vi "Dresden R2R Sputter 03.02.2018 IY24.vi"() -> ()   [LabVIEW 2009] (continued)
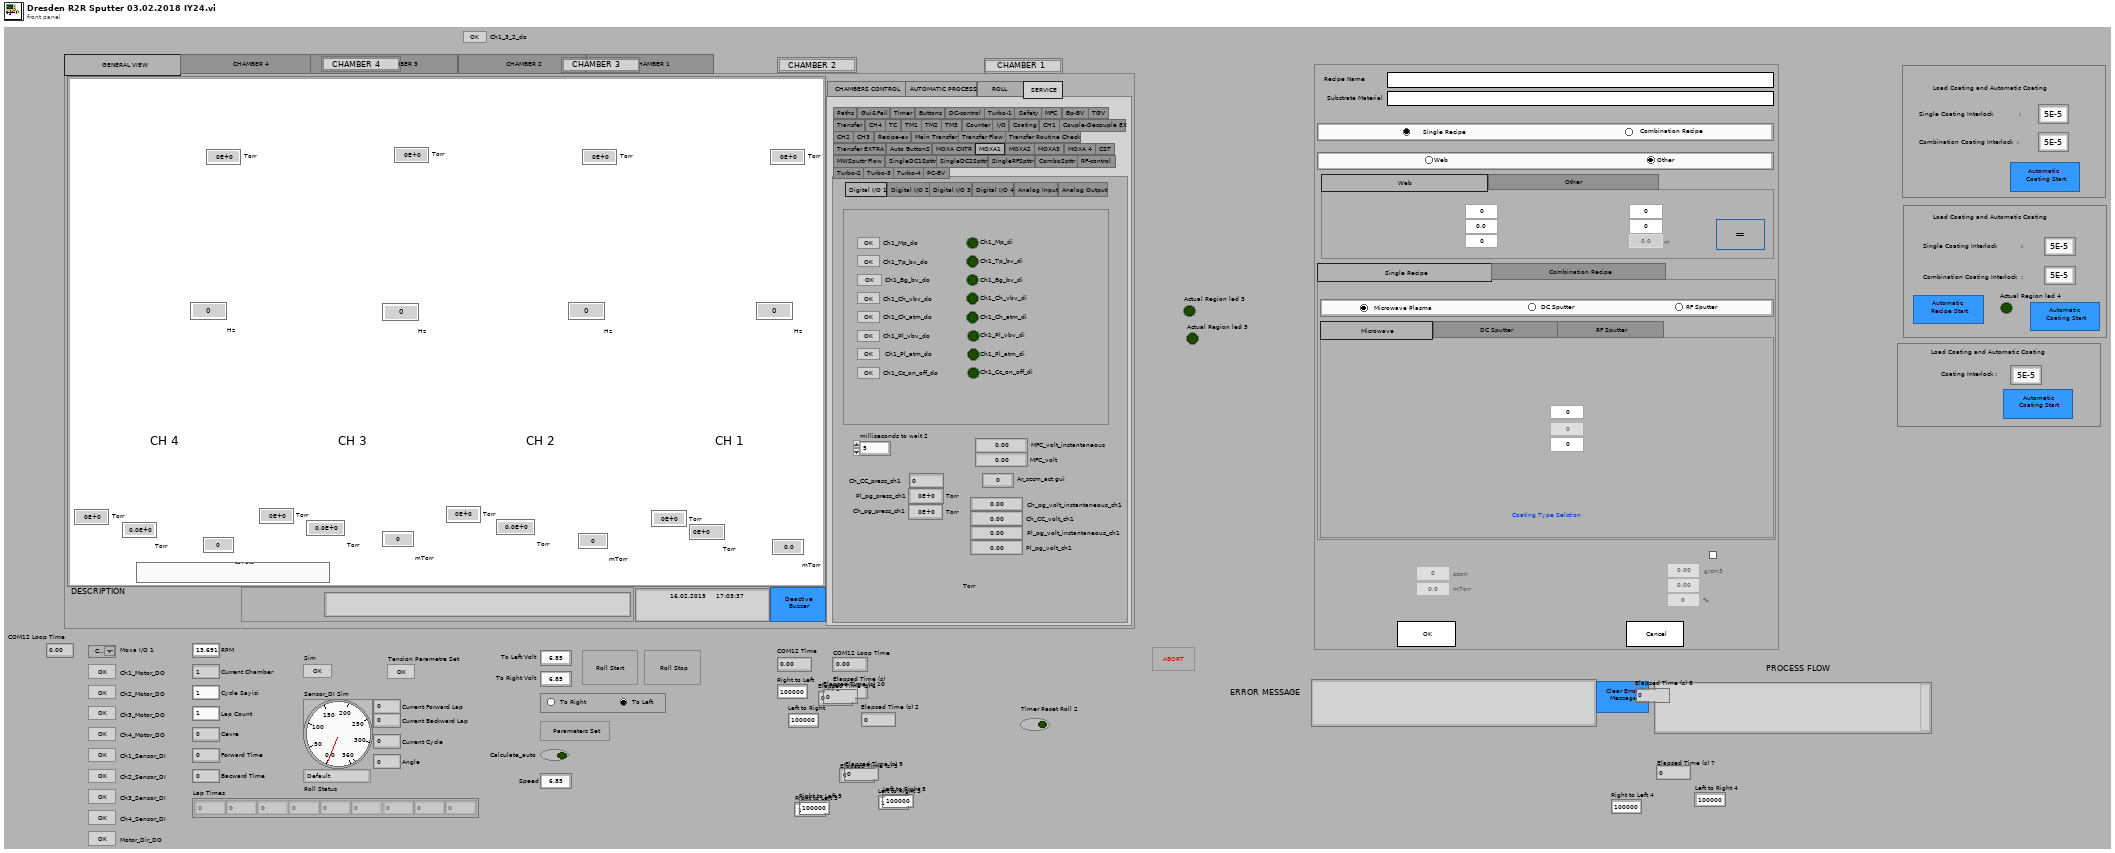
[diagram p1: front panel]
types:
  T1 = typedef "Roll_StatusT.ctl" = enum16{"Default", "Initiate", "Transfer", "Start", "Home", "HomeP", "Forward", "Pause", "Backward", "Stop", "Security"}
  T2 = enum32{"Single Recipe                                                                         ", "Combination Recipe                                                              "}
  T3 = enum32{"Microwave Plasma", "DC Sputter", "RF Sputter"}
  T4 = enum32{"Microwave                                          ", "DC Sputter                                                 ", "RF Sputter                                       "}
  T5 = enum32{"Web                                                                                    ", "Other                                                                                    "}
  T6 = enum32{"  GENERAL VIEW                                   ", "     CHAMBER 4                                             ", "              CHAMBER 3                                              ", " CHAMBER 2                                                ", " CHAMBER 1                                                "}
  T7 = enum32{"CHAMBERS CONTROL    ", "AUTOMATIC PROCESS", "ROLL             ", "SERVICE    "}
  T8 = enum32{"CHAMBER 4      ", "CHAMBER 3       ", "CHAMBER 2       ", "CHAMBER 1         "}
  T9 = enum32{"PUMP & SHUTDOWN CONTROL               ", "PROCESS FLOW                    "}
  T10 = enum32{"Pumping(ch4>0.9 torr)", "Pumping(ch4<0.9 torr)", "Shut Down "}
  T11 = enum32{"Pumping(ch3>0.9 torr)", "Pumping(ch3<0.9 torr)   ", "Shut Down       "}
  T12 = enum32{"Pumping(CH2>0.9 Torr)     ", "Pumping(ch2<0.9 torr)", "Shut Down    "}
  T13 = enum32{"Pumping(CH1>0.9 Torr ", "Pumping(CH1<0.9Torr)    ", "Shut Down       "}
  T14 = enum32{"Chamber I", "Chamber 2", "Chamber 3", "Chamber 4"}
  T15 = enum32{"Full Foil              ", "Specified Length of Foil "}
  T16 = enum32{"Left to Right                ", "Right to Left                  "}
  T17 = enum32{"Paths", "Gui&Fail", "Timer", "Buttons", "DC-control", "Turbo-1", "Safety", "MFC", "Bp-BV", "TGV", "Transfer", "CH4", "TC", "TM1", "TM2", "TM3", "Counter", "I/O", "Coating", "CH1", "Couple-Decouple EX", "CH2", "CH3", "Recipe-ex", "Main Transfer", "Transfer Flow", "Transfer Routine Check", "Transfer EXTRA", "Auto ButtonS", "MOXA CNTR", "MOXA1", "MOXA2", "MOXA3", "MOXA 4", "CST", "MWSputtr Flow", "SingleDC1Spttr", "SingleDC2Spttr", "SingleRFSpttr", "ComboSpttr", "RF-control", "Turbo-2", "Turbo-3", "Turbo-4", "PC-BV"}
  T18 = enum32{"    Page 1        ", "      Page 2        ", "         Page 3        "}
  T19 = enum32{"             Page 1            ", "           Page 2            ", "          Page 3           "}
  T20 = enum32{"Paths", "Gui&fail", "Timer", "Moxa-Ch4", "Buttons", "Automatic Procedure Process Flow", "Auto Pump", "Auto Shutdown", "Transfer4_3"}
  T21 = enum32{"TC1", "TC 2", "Rolling Parameters", "Test"}
  T22 = enum32{"Paths", "Gu&Fail", "Timer", "Moxa-Ch1", "Buttons", "Auto Pump", "Auto shutdown"}
  T23 = enum32{"Paths", "Gui&Fail", "Timer", "Moxa-Ch2", "Buttons", "Auto Pump", "Auto shutdown", "transfer2-3"}
  T24 = enum32{"Paths", "Gui&Fail", "Timer", "Moxa-Ch2", "Buttons", "Auto Pump", "Auto Shut Down", "transfer"}
  T25 = enum32{"Transfer CH1-CH2", "Transfer CH2-CH3 ", "Transfer CH3-CH4", "Transfer CH2-CH1", "Transfer CH3-CH2", "Transfer CH4-CH3"}
  T26 = enum32{"Digital I/O 1", "Digital I/O 2", "Analog Output"}
  T27 = enum32{"Digital I/O 1", "Digital I/O 2", "Digital I/O 3", "Digital I/O 4", "Analog Input", "Analog Output"}
  T28 = enum32{"MANUAL RF COATING CONTROL                                         "}
  T29 = enum32{"RF Power Supply Control", "  Ramp Timer", "Pulsing ", "Capacitor"}
  T30 = enum32{"MANUAL DC COATING CONTROL                                   ..."}
  T31 = enum32{"DC Power Supply Control           ", "Ramp Timer                "}
  T32 = enum32{"DC Power Supply Control   ", "Ramp Timer                     "}
  T33 = enum32{"MANUAL MICROWAVE PLASMA CONTROL                            "}
  T34 = typedef "imagedata.ctl" = cluster{"image type":i32, "image depth":i32, "image":u8[], "mask":u8[], "colors":u32[], "Rectangle":cluster{"left":i16, "top":i16, "right":i16, "bottom":i16}}
  T35 = cluster{"Font Name:":string, "Size":i16, "Strikeout?":bool, "Italic?":bool, "Underline?":bool, "Outline?":bool, "Shadow?":bool, "Bold?":bool}
  T36 = enum16{"User-specified Font", "Application Font", "System Font", "Dialog Font"}
  T37 = typedef "LVMouseTypeDef.ctl" = cluster{"Mouse Position":cluster{"X":i32, "Y":i32}, "Mouse Modifiers":cluster{"Button Down":bool, "Shift Mod":bool, "Menu Mod":bool, "Option Mod":bool}}
  T38 = cluster{"Button Down":bool, "Shift Mod":bool, "Menu Mod":bool, "Option Mod":bool}
  T39 = cluster{"Mode":enum16{"RTU", "ASCII"}, "Slave Address":u8}
  T40 = enum16{"Left Button", "Center Button", "Right Button", "Window Close"}
diagram:
  w2 = data[3B] items=["Default", "Initiate", "Transfer", "Start", "Home", "HomeP", "Forward", "Pause", "Backward", "Stop", "Security"] ("Roll Status")
  w22 = data[3B] items=["RTU", "ASCII"] ("Mode")
  w20 = data[3B] items=["None", "Odd", "Even", "Mark", "Space"] ("Parity")
  (unwired) i32? 19200 ("Baud Rate")
  w28 = data[3B] items=["RTU", "ASCII"] ("Mode")
  w30 = data[3B] items=["None", "Odd", "Even", "Mark", "Space"] ("Parity")
  w750 = data[3B] items=["RTU", "ASCII"] ("Mode")
  w752 = data[3B] items=["None", "Odd", "Even", "Mark", "Space"] ("Parity")
  w766 = data[3B] items=["RTU", "ASCII"] ("Mode")
  w764 = data[3B] items=["None", "Odd", "Even", "Mark", "Space"] ("Parity")
  w767 = data[3B] items=["RTU", "ASCII"] ("Mode")
  w769 = data[3B] items=["None", "Odd", "Even", "Mark", "Space"] ("Parity")
  w780 = data[3B] items=["RTU", "ASCII"] ("Mode")
  w778 = data[3B] items=["None", "Odd", "Even", "Mark", "Space"] ("Parity")
  w787 = data[3B] items=["RTU", "ASCII"] ("Mode")
  w785 = data[3B] items=["None", "Odd", "Even", "Mark", "Space"] ("Parity")
  w792 = data[3B] items=["RTU", "ASCII"] ("Mode")
  w794 = data[3B] items=["None", "Odd", "Even", "Mark", "Space"] ("Parity")
  w821 = i16? 1 items=["None", "Odd", "Even", "Mark", "Space"] ("parity (0:none)")
  w825 = i16? 2 items=["None", "Odd", "Even", "Mark", "Space"] ("parity (0:none)")
  w834 = i16? 1 items=["None", "Odd", "Even", "Mark", "Space"] ("parity (0:none)")
  # "Timer"
  # "Elapsed Time Array"
  # "Status"
  # "Chamber No"
  # "*Initiate\nAmac: Baslangic degerlerinin okuyor ve start val bekliyor.\nBulundugu camber degerini okuyor. (1-4)\nLap sayisini okuyor.\nCycle sayisini okuyor.\n\nSistem hep soldan saga sarma yapabiliyor.\n\nStart val degerini okuyan loop yapıyor.\nStart val 1 olmasi ile Start state'e gidiyor.\n\n*Start State\nAmac: Motoru calıstırmak. \nMotoru Calistiriyor.\nHome state'e gidiyor.\n\n*Home State\nAmac: Belirli bir ref noktadan prosesi baslatmak.\nTam dolu yarim aya girince baslatir.\nDolu yarim aya girince forward state'e gidiyor.\nForward Timer baslatilir.\n\n*Forward State\nBaslangicta dolu yarim ayin basindan sonuna ilerler ve bosa cikar.\nIlk tur icinde once bosa cikar ve\nDolu yarim aya tekrar girince tur atmis olur.\nTur atlayinca Lap Sayisini 1 azaltir. Back Lap sayisini 1 arttirir.\nBack tur sayisi ilk tur ile birlikte 2 olur. Cunku Geri gidiste, \ntur atmadan ilk bosa dususu kompanse etmek gerekmektedir.\nLap sayisi kalan degeri 0 olunca Pause State'e gider.\nLap Times'a Forward Lap Time kayit edilir.\n\n*Backward State\nBaslangicta dolu yarim ayin hemen basindan geri gider ve bosa cikar,\nİlk bosa cikis tam tur olmadigindan deger back tur degeri 2 den 1 olur.\nIlk tur icinde once bosata ilerler ve dolu tarafa gecer.\nDolu yarim ay tekrar bitince geri tur atmis olur.\nTur atlayinca Back Lap sayisini 1 azalir.\nBack Lap sayisi kalan degeri 0 olunca Cycle degeri 1 azalir.\nCycle sayisi degeri 0 olursa Stop State'e yoksa Pause State'e gider.\nLap Times'a Backward Lap Time kayit edilir.\n\n*Pause State\nMotorlarin tamamina dur komutu yollanir.\n1 saniye beklenir.\nYon degistirilir.\nLap Times'a Pause yi gosteren 0 degeri kayit edilir.\nTension Parametre Set Yollanir.\nMotor calıstırılır.\nBackward veya Forward Timer baslatilir."
  # "Moxa R1212 uzerinde \nDI starting adresi 0 ve quantity 16 adet yapılabilir.\nDO starting adres 320 ve quantity girmeye gerekyok.\n\nMoxa manuelinde \n1 nolu adres DI0 value demek.\n321 nolu adres DO_0 value demek.\nLabview, Manuele adresinden 1 eksik degerler istiyor.\n \nVaksis programlarında DI starting adres 8 olarak secilmis. (8 secilmesinin nedeni ilk 8 adresin jumperlar ile DO DI yapilabilir adresler olmasi ve bunların DO olarak kullanılması olabilir.)"
  # "Moxa R1212 uzerinde \n8 adet DI \n8 adet DO bulunmaktadir. \nDO jumper ile DI'ye donusturulebilmektedir."
  # "Back Tur"
  # "Cycle"
  # "Forward Tur"
  # "Speed"
  # "right to left 4/5 true 2/2 actual region led"
  # "Gui & Text"
  # "Digital & Analog Inputs / Outputs"
  # "TRANSFER PROCESS"
  n1 = while {
    stop <- FALSE stop-if-true
    n2 = Wait Until Next ms Multiple(millisecond multiple=u32 300) -> ()  [unwired: 1 out]
    n3 = local read "Start_up_ch2"() -> (w852:bool)
    n4 = local read "Start_up_ch3"() -> (w847:bool)
    n5 = local read "Start_up_ch4"() -> (w844:bool)
    n6 = local read "Start_up_ch1"() -> (w855:bool)
    n7 = case shown="True" w852 {
      frame #0 {
      }
      frame #1 {
        n8 = local read "Ch2_pressure2"() -> (→"Pressure_time_graph_ch2":dbl)
        n9 = Wait (ms)(milliseconds to wait=u32 1000) -> ()  [unwired: 1 out]
      }
    }
    n10 = case shown="True" w847 {
      frame #0 {
      }
      frame #1 {
        n11 = local read "Ch3_pressure2"() -> (→"Pressure_time_graph_ch3":dbl)
        n12 = Wait (ms)(milliseconds to wait=u32 1000) -> ()  [unwired: 1 out]
      }
    }
    n13 = case shown="True" w844 {
      frame #0 {
      }
      frame #1 {
        n14 = local read "Ch4pressure"() -> (→"Pressure_time_graph_ch4":dbl)
        n15 = Wait (ms)(milliseconds to wait=u32 1000) -> ()  [unwired: 1 out]
      }
    }
    n16 = case shown="True" w855 {
      frame #0 {
      }
      frame #1 {
        n17 = local read "Ch1_pressure 2"() -> (→"Pressure_time_graph_ch1":dbl)
        n18 = Wait (ms)(milliseconds to wait=u32 1000) -> ()  [unwired: 1 out]
      }
    }
    n19 = feedback #1() -> (w851:bool)  [unwired: 1 in]
    n20 = feedback #2() -> (w856:bool)  [unwired: 1 in]
    n21 = feedback #3() -> (w848:bool)  [unwired: 1 in]
    n22 = feedback #4() -> (w843:bool)  [unwired: 1 in]
    n23 = case shown="True" w852 {
      tunnel: [TRUE FALSE] -> w850
      tunnel: w851 -> [_ w904]
      frame #0 {
      }
      frame #1 {
        n24 = call "Elapsed Time126"("Reset"=w904) -> ("Elapsed Time (s)"=→"Auto_pump_time_ch2" →"Graph_pumping_time_ch2":dbl)  [unwired: 11 in, 7 out]
      }
    }
    n25 = case shown="True" w855 {
      tunnel: [TRUE FALSE] -> w857
      tunnel: w856 -> [_ w920]
      frame #0 {
      }
      frame #1 {
        n26 = call "Elapsed Time101"("Reset"=w920) -> ("Elapsed Time (s)"=→"Auto_pump_time_ch1" →"Graph_pumping_time_ch1":dbl)  [unwired: 11 in, 7 out]
      }
    }
    n27 = case shown="True" w847 {
      tunnel: [TRUE FALSE] -> w849
      tunnel: w848 -> [_ w888]
      frame #0 {
      }
      frame #1 {
        n28 = call "Elapsed Time128"("Reset"=w888) -> ("Elapsed Time (s)"=→"Auto_pump_time_ch3" →"Graph_pumping_time_ch3":dbl)  [unwired: 11 in, 7 out]
      }
    }
    n29 = case shown="True" w844 {
      tunnel: [TRUE FALSE] -> w842
      tunnel: w843 -> [_ w872]
      frame #0 {
      }
      frame #1 {
        n30 = call "Elapsed Time137"("Reset"=w872) -> ("Elapsed Time (s)"=→"Auto_pump_time_ch4" →"Graph_pumping_time_ch4":dbl)  [unwired: 11 in, 7 out]
      }
    }
    n31 = case shown="True" w852 {
      frame #0 {
      }
      frame #1 {
        n32 = local read "Graph_pumping_time_ch2"() -> (w899:dbl)
        n33 = Divide(x=w899, y=60.0 ("X Scale.Range:Maximum")) -> (x/y=w900:dbl)
        n34 = Increment(x=w900) -> (x+1=w898:dbl)
        n35 = property on="Pressure_time_graph_ch2" class="WFChart (strict)"("XScale.Maximum"=w898, "XScale.Minimum"=0.0 ("X Scale.Range:Minimum")) -> ()  [unwired: 2 in, 2 out]
        n36 = property on="Pressure_time_graph_ch2" class="WFChart (strict)"("YScale.Maximum"=1000.0 ("Y Scale.Range:Maximum"), "YScale.Minimum"=5e-08 ("Y Scale.Range:Minimum")) -> ()  [unwired: 2 in, 2 out]
        n37 = property on="Pressure_time_graph_ch2" class="WFChart (strict)"("XScale.Multiplier"=0.0166 ("X Scale.Offset and Multiplier:Multiplier 2")) -> ()  [unwired: 2 in, 2 out]
      }
    }
    n38 = case shown="True" w855 {
      frame #0 {
      }
      frame #1 {
        n39 = local read "Graph_pumping_time_ch1"() -> (w915:dbl)
        n40 = Divide(x=w915, y=60.0 ("X Scale.Range:Maximum")) -> (x/y=w916:dbl)
        n41 = Increment(x=w916) -> (x+1=w914:dbl)
        n42 = property on="Pressure_time_graph_ch1" class="WFChart (strict)"("XScale.Maximum"=w914, "XScale.Minimum"=0.0 ("X Scale.Range:Minimum")) -> ()  [unwired: 2 in, 2 out]
        n43 = property on="Pressure_time_graph_ch1" class="WFChart (strict)"("YScale.Maximum"=1000.0 ("Y Scale.Range:Maximum"), "YScale.Minimum"=5e-08 ("Y Scale.Range:Minimum")) -> ()  [unwired: 2 in, 2 out]
        n44 = property on="Pressure_time_graph_ch1" class="WFChart (strict)"("XScale.Multiplier"=0.0166 ("X Scale.Offset and Multiplier:Multiplier 2")) -> ()  [unwired: 2 in, 2 out]
      }
    }
    n45 = case shown="True" w847 {
      frame #0 {
      }
      frame #1 {
        n46 = local read "Graph_pumping_time_ch3"() -> (w883:dbl)
        n47 = Divide(x=w883, y=60.0 ("X Scale.Range:Maximum")) -> (x/y=w884:dbl)
        n48 = Increment(x=w884) -> (x+1=w882:dbl)
        n49 = property on="Pressure_time_graph_ch3" class="WFChart (strict)"("XScale.Maximum"=w882, "XScale.Minimum"=0.0 ("X Scale.Range:Minimum")) -> ()  [unwired: 2 in, 2 out]
        n50 = property on="Pressure_time_graph_ch3" class="WFChart (strict)"("YScale.Maximum"=1000.0 ("Y Scale.Range:Maximum"), "YScale.Minimum"=5e-08 ("Y Scale.Range:Minimum")) -> ()  [unwired: 2 in, 2 out]
        n51 = property on="Pressure_time_graph_ch3" class="WFChart (strict)"("XScale.Multiplier"=0.0166 ("X Scale.Offset and Multiplier:Multiplier 2")) -> ()  [unwired: 2 in, 2 out]
      }
    }
    n52 = case shown="True" w844 {
      frame #0 {
      }
      frame #1 {
        n53 = local read "Graph_pumping_time_ch4"() -> (w867:dbl)
        n54 = Divide(x=w867, y=60.0 ("X Scale.Range:Maximum")) -> (x/y=w868:dbl)
        n55 = Increment(x=w868) -> (x+1=w866:dbl)
        n56 = property on="Pressure_time_graph_ch4" class="WFChart (strict)"("XScale.Maximum"=w866, "XScale.Minimum"=0.0 ("X Scale.Range:Minimum")) -> ()  [unwired: 2 in, 2 out]
        n57 = property on="Pressure_time_graph_ch4" class="WFChart (strict)"("YScale.Maximum"=1000.0 ("Y Scale.Range:Maximum"), "YScale.Minimum"=5e-08 ("Y Scale.Range:Minimum")) -> ()  [unwired: 2 in, 2 out]
        n58 = property on="Pressure_time_graph_ch4" class="WFChart (strict)"("XScale.Multiplier"=0.0166 ("X Scale.Offset and Multiplier:Multiplier 2")) -> ()  [unwired: 2 in, 2 out]
      }
    }
    n59 = case shown="True" "Show_graph_ch2" {
      frame #0 {
        n60 = property on="Graph_tab_ch2" class="TabCtl (strict)"("Visible"=TRUE) -> ()  [unwired: 2 in, 2 out]
      }
      frame #1 {
        n61 = property on="Graph_tab_ch2" class="TabCtl (strict)"("Visible"=FALSE) -> ()  [unwired: 2 in, 2 out]
      }
    }
    n62 = case shown="True" "Show_graph_ch1" {
      frame #0 {
        n63 = property on="Graph_tab_ch1" class="TabCtl (strict)"("Visible"=TRUE) -> ()  [unwired: 2 in, 2 out]
      }
      frame #1 {
        n64 = property on="Graph_tab_ch1" class="TabCtl (strict)"("Visible"=FALSE) -> ()  [unwired: 2 in, 2 out]
      }
    }
    n65 = case shown="True" "Show_graph_ch3" {
      frame #0 {
        n66 = property on="Graph_tab_ch3" class="TabCtl (strict)"("Visible"=TRUE) -> ()  [unwired: 2 in, 2 out]
      }
      frame #1 {
        n67 = property on="Graph_tab_ch3" class="TabCtl (strict)"("Visible"=FALSE) -> ()  [unwired: 2 in, 2 out]
      }
    }
    n68 = case shown="True" "Show_graph_ch4" {
      frame #0 {
        n69 = property on="Graph_tab_ch4" class="TabCtl (strict)"("Visible"=TRUE) -> ()  [unwired: 2 in, 2 out]
      }
      frame #1 {
        n70 = property on="Graph_tab_ch4" class="TabCtl (strict)"("Visible"=FALSE) -> ()  [unwired: 2 in, 2 out]
      }
    }
  }
  n71 = while {
    stop <- FALSE stop-if-true
    n72 = local read "Semi"() -> (w924:bool)
    n73 = Wait Until Next ms Multiple(millisecond multiple=u32 300) -> ()  [unwired: 1 out]
    n74 = feedback #5() -> (w926:bool)  [unwired: 1 in]
    n75 = case shown="True" w924 {
      tunnel: w926 -> [_ w946]
      tunnel: [TRUE FALSE] -> w925
      frame #0 {
      }
      frame #1 {
        w930 = FALSE
        w932 = FALSE
        n76 = call "Elapsed Time99"("Reset"=w946) -> ("Elapsed Time (s)"=w933:dbl)  [unwired: 11 in, 7 out]
        n77 = In Range and Coerce(upper limit=2.3, x=w933, lower limit=2.0) -> (In Range?=w943:bool)  [unwired: 1 out]
        n78 = In Range and Coerce(upper limit=4.3, x=w933, lower limit=4.0) -> (In Range?=w942:bool)  [unwired: 1 out]
        n79 = In Range and Coerce(upper limit=6.3, x=w933, lower limit=6.0) -> (In Range?=w937:bool)  [unwired: 1 out]
        n80 = In Range and Coerce(upper limit=11.3, x=w933, lower limit=11.0) -> (In Range?=w936:bool)  [unwired: 1 out]
        n81 = In Range and Coerce(upper limit=0.3, x=w933, lower limit=0.0) -> (In Range?=w931:bool)  [unwired: 1 out]
        n82 = disable-structure shown="Disabled" {
          disable-tunnel: w943 -> [w953 _]
          disable-tunnel: w942 -> [w952 _]
          disable-tunnel: w937 -> [w951 _]
          disable-tunnel: w931 -> [w950 _]
          frame #0 {
            n83 = case shown="True" w950 {
              frame #0 {
              }
              frame #1 {
                w958 = FALSE
                w959 = FALSE
                w960 = FALSE
                w961 = TRUE
                w962 = FALSE
                w963 = TRUE
                w964 = TRUE ("Cnt_Do_Buzzer")
                w965 = FALSE
                n84 = local write "Casette_servo_start/stop_do"(w965) -> ()
                n85 = local write "Tension_controllers_start/stop_do"(w965) -> ()
                n86 = local write "Security_cancel_ch1"(w963) -> ()
                n87 = local write "Security_cancel_ch2"(w963) -> ()
                n88 = local write "Security_cancel_ch3"(w963) -> ()
                n89 = local write "Security_cancel_ch4"(w963) -> ()
                n90 = local write "Ch1_Tp_bv_do"(w962) -> ()
                n91 = local write "Ch1_Bg_bv_do"(w962) -> ()
                n92 = local write "Ch1_Ch_vbv_do"(w962) -> ()
                n93 = local write "Ch1_Pl_vbv_do"(w962) -> ()
                n94 = local write "Ch1_Cc_on_off_do"(w962) -> ()
                n95 = local write "Ch1_Sov_Ar_do"(w962) -> ()
                n96 = local write "Ch1_SRV_start_stop_do"(w962) -> ()
                n97 = local write "Ch1_TGV_control_do"(w962) -> ()
                n98 = local write "Pc_bv1_auto_close"(w961) -> ()
                n99 = local write "Tp1_auto_stop"(w961) -> ()
                n100 = local write "Ch3_Tp_bv_do"(w959) -> ()
                n101 = local write "Ch3_Bg_bv_do"(w959) -> ()
                n102 = local write "Ch3_Ch_vbv_do"(w959) -> ()
                n103 = local write "Ch3_Pl_vbv_do"(w959) -> ()
                n104 = local write "Ch3_Cc_on_off_do"(w959) -> ()
                n105 = local write "Ch3_Sov_Ar_do"(w959) -> ()
                n106 = local write "Ch3_SRV_start_stop_do"(w959) -> ()
                n107 = local write "Ch3_TGV_control_do"(w959) -> ()
                n108 = local write "Cnt_Do_Buzzer"(w964) -> ()
                n109 = local write "Ar_auto_set_zero_ch1"(w964) -> ()
                n110 = local write "Dc_auto_off"(w964) -> ()
                n111 = local write "RF_auto_off"(w964) -> ()
                n112 = local write "MW1_off"(w964) -> ()
                n113 = local write "Test_stop"(w964) -> ()
                n114 = local write "Ch2_Tp_bv_do"(w960) -> ()
                n115 = local write "Ch2_Bg_bv_do"(w960) -> ()
                n116 = local write "Ch2_Ch_vbv_do"(w960) -> ()
                n117 = local write "Ch2_Pl_vbv_do"(w960) -> ()
                n118 = local write "Ch2_Cc_on_off_do"(w960) -> ()
                n119 = local write "Ch2_Sov_Ar_do"(w960) -> ()
                n120 = local write "Ch2_SRV_start_stop_do"(w960) -> ()
                n121 = local write "Ch2_TGV_control_do"(w960) -> ()
                n122 = local write "Ch4_Tp_bv_do"(w958) -> ()
                n123 = local write "Ch4_Bg_bv_do"(w958) -> ()
                n124 = local write "Ch4_Ch_vbv_do"(w958) -> ()
                n125 = local write "Ch4_Pl_vbv_do"(w958) -> ()
                n126 = local write "Ch4_Cc_on_off_do"(w958) -> ()
                n127 = local write "Ch4_Sov_Ar_do"(w958) -> ()
                n128 = local write "Ch4_SRV_start_stop_do"(w958) -> ()
                n129 = local write "Ch4_TGV_control_do"(w958) -> ()
              }
            }
            n130 = case shown="True" w952 {
              frame #0 {
              }
              frame #1 {
                w954 = TRUE
                n131 = local write "Pc_bv3_auto_close"(w954) -> ()
                n132 = local write "Tp3_auto_stop"(w954) -> ()
              }
            }
            n133 = case shown="True" w951 {
              frame #0 {
              }
              frame #1 {
                w966 = TRUE
                n134 = local write "Pc_bv4_auto_close"(w966) -> ()
                n135 = local write "Tp4_auto_stop"(w966) -> ()
              }
            }
            n136 = case shown="True" w953 {
              frame #0 {
              }
              frame #1 {
                w955 = TRUE
                w957 = TRUE
                w956 = FALSE
                n137 = local write "Cnt_Dcps_sw1_do"(w956) -> ()
                n138 = local write "Cnt_Dcps_sw2_do"(w956) -> ()
                n139 = local write "Ar_auto_set_zero_ch3"(w957) -> ()
                n140 = local write "MW2_off"(w957) -> ()
                n141 = local write "Pc_bv2_auto_close"(w955) -> ()
                n142 = local write "Tp2_auto_stop"(w955) -> ()
              }
            }
          }
          frame #1 {
          }
        }
        n143 = case shown="True" w936 {
          frame #0 {
          }
          frame #1 {
            w968 = FALSE
            n144 = local write "Security_cancel_ch1"(w968) -> ()
            n145 = local write "Security_cancel_ch2"(w968) -> ()
            n146 = local write "Security_cancel_ch3"(w968) -> ()
            n147 = local write "Security_cancel_ch4"(w968) -> ()
            n148 = local write "Cnt_Do_Buzzer"(w968) -> ()
            n149 = local write "Semi"(w968) -> ()
            n150 = local write "Statue_abort"(w968) -> ()
          }
        }
        n151 = case shown="True" w931 {
          frame #0 {
          }
          frame #1 {
            n152 = local write "Cnt_Do_Buzzer"(TRUE ("Cnt_Do_Buzzer")) -> ()
          }
        }
        n153 = local write "Routine_check_transfer"(w932) -> ()
        n154 = local write "Transfer_ch1_2"(w932) -> ()
        n155 = local write "Transfer_ch2_1"(w932) -> ()
        n156 = local write "Transfer_ch2_3"(w932) -> ()
        n157 = local write "Transfer_ch3_2"(w932) -> ()
        n158 = local write "Transfer_ch3_4"(w932) -> ()
        n159 = local write "Transfer_ch3_4"(w932) -> ()
        n160 = local write "Start_up_ch1"(w932) -> ()
        n161 = local write "Start_up_ch2"(w932) -> ()
        n162 = local write "Start_up_ch3"(w932) -> ()
        n163 = local write "Start_up_ch4"(w932) -> ()
        n164 = local write "Shutdown_ch1"(w932) -> ()
        n165 = local write "Shutdown_ch2"(w932) -> ()
        n166 = local write "Shutdown_ch3"(w932) -> ()
        n167 = local write "Shutdown_ch4"(w932) -> ()
        n168 = local write "Start_coating"(w932) -> ()
        n169 = local write "Start_Coating_MW"(w932) -> ()
        n170 = local write "Start_Coating_Ch4"(w932) -> ()
        n171 = local write "Start_Coating_Ch2"(w932) -> ()
        n172 = local write "Start_Coating_Ch3"(w932) -> ()
        n173 = local write "Casette_servo_start/stop_do"(w930) -> ()
        n174 = local write "Tension_controllers_start/stop_do"(w930) -> ()
        n175 = local write "Automatic Roll"(w930) -> ()
      }
    }
  }
  n176 = stacked-sequence {
    frame #0 {
    }
  }
  n177 = local write "Ch2_TGV_control_do"(T/1 ("Ch2_TGV_control_do")) -> ()
  n178 = stacked-sequence {
    frame #0 {
      w969 = ""
      "Error Message" <- w969
      "system_status" <- "Semi-automatic is active" ("system_statu")
      "final_process_messages" <- w969
    }
  }
  n179 = stacked-sequence {
    frame #0 {
      # "OTHER  BUTTONS"
      n180 = while {
        stop <- i16? 0 stop-if-true
        # "OPEN/CLOSE & START &STOP"
        n181 = stacked-sequence {
          frame #0 {
            n182 = Or(x="Ch1_Mp_start_gui", y="Ch1_Mp_start") -> (x .or. y?=w1776)
            n183 = Or(x="Ch1_Mp_stop_gui", y="Ch1_Mp_stop") -> (x .or. y?=w1775)
            n184 = case shown="True" w1775 {
              frame #0 {
              }
              frame #1 {
                n185 = local read "Ch1_Mp_stop_safety"() -> (w1819)
                n186 = case shown="True" w1819 {
                  frame #0 {
                    n187 = local write "Error Message"("MP can not be stopped.\nReason :                           \n*TP-BV can be open.       " ("Error Message")) -> ()
                  }
                  frame #1 {
                    n188 = stacked-sequence {
                      frame #0 {
                        n189 = local write "Ch1_Mp_do"(i16? 0 ("Ch1_Mp_do")) -> ()
                      }
                      frame #1 {
                        n190 = Wait (ms)(milliseconds to wait=i32? 500) -> ()  [unwired: 1 out]
                      }
                      frame #2 {
                        n191 = local write "Ch1_Pl_atm_do"(i16? 0 ("Ch1_Mp_do")) -> ()
                      }
                      frame #3 {
                        n192 = Wait (ms)(milliseconds to wait=i32? 500) -> ()  [unwired: 1 out]
                      }
                      frame #4 {
                        n193 = local write "Ch1_Pl_vbv_do"(T/1 ("Ch1_Pl_vbv_do")) -> ()
                      }
                    }
                  }
                }
              }
            }
            n194 = case shown="True" w1776 {
              frame #0 {
              }
              frame #1 {
                n195 = local read "Ch1_Mp_start_safety"() -> (w1826)
                n196 = case shown="True" w1826 {
                  frame #0 {
                    n197 = local write "Error Message"("MP can not be started.\nReason:                          \n*PL-VBV can be open. \n   *CH-VBV can be open." ("Error Message")) -> ()
                  }
                  frame #1 {
                    n198 = stacked-sequence {
                      frame #0 {
                        n199 = local write "Ch1_Pl_atm_do"(T/1 ("Ch1_Mp_do")) -> ()
                      }
                      frame #1 {
                        n200 = Wait (ms)(milliseconds to wait=i32? 1000) -> ()  [unwired: 1 out]
                      }
                      frame #2 {
                        n201 = local write "Ch1_Ch_atm_do"(T/1 ("Ch1_Mp_do")) -> ()
                      }
                      frame #3 {
                        n202 = Wait (ms)(milliseconds to wait=i32? 1000) -> ()  [unwired: 1 out]
                      }
                      frame #4 {
                        n203 = local write "Ch1_Mp_do"(T/1 ("Ch1_Mp_do")) -> ()
                      }
                    }
                  }
                }
              }
            }
            n204 = Or(x="Ch2_Mp_start_gui", y="Ch2_Mp_start") -> (x .or. y?=w1773)
            n205 = Or(x="Ch2_Mp_stop_gui", y="Ch2_Mp_stop") -> (x .or. y?=w1774)
            n206 = case shown="True" w1773 {
              frame #0 {
              }
              frame #1 {
                n207 = local read "Ch2_Mp_start_safety"() -> (w1812)
                n208 = case shown="True" w1812 {
                  frame #0 {
                    n209 = local write "Error Message"("MP can not be started.\nReason:*PL-VBV can be open. \n   *CH-VBV can be open." ("Error Message")) -> ()
                  }
                  frame #1 {
                    n210 = stacked-sequence {
                      frame #0 {
                        n211 = local write "Ch2_Pl_atm_do"(T/1 ("Ch1_Mp_do")) -> ()
                      }
                      frame #1 {
                        n212 = Wait (ms)(milliseconds to wait=i32? 1000) -> ()  [unwired: 1 out]
                      }
                      frame #2 {
                        n213 = local write "Ch2_Ch_atm_do"(T/1 ("Ch1_Mp_do")) -> ()
                      }
                      frame #3 {
                        n214 = Wait (ms)(milliseconds to wait=i32? 1000) -> ()  [unwired: 1 out]
                      }
                      frame #4 {
                        n215 = local write "Ch2_Mp_do"(T/1 ("Ch1_Mp_do")) -> ()
                      }
                    }
                  }
                }
              }
            }
            n216 = case shown="True" w1774 {
              frame #0 {
              }
              frame #1 {
                n217 = local read "Ch2_Mp_stop_safety"() -> (w1805)
                n218 = case shown="True" w1805 {
                  frame #0 {
                    n219 = local write "Error Message"("MP can not be stopped.\nReason :*TP-BV can be open." ("Error Message")) -> ()
                  }
                  frame #1 {
                    n220 = stacked-sequence {
                      frame #0 {
                        n221 = local write "Ch2_Mp_do"(i16? 0 ("Ch1_Mp_do")) -> ()
                      }
                      frame #1 {
                        n222 = Wait (ms)(milliseconds to wait=i32? 500) -> ()  [unwired: 1 out]
                      }
                      frame #2 {
                        n223 = local write "Ch2_Pl_atm_do"(i16? 0 ("Ch1_Mp_do")) -> ()
                      }
                      frame #3 {
                        n224 = Wait (ms)(milliseconds to wait=i32? 500) -> ()  [unwired: 1 out]
                      }
                      frame #4 {
                        n225 = local write "Ch2_Pl_vbv_do"(T/1 ("Ch1_Pl_vbv_do")) -> ()
                      }
                    }
                  }
                }
              }
            }
            n226 = Or(x="Ch3_Mp_stop_gui", y="Ch3_Mp_stop") -> (x .or. y?=w1771)
            n227 = Or(x="Ch3_Mp_start_gui", y="Ch3_Mp_start") -> (x .or. y?=w1772)
            n228 = case shown="True" w1772 {
              frame #0 {
              }
              frame #1 {
                n229 = local read "Ch3_Mp_start_safety"() -> (w1798)
                n230 = case shown="True" w1798 {
                  frame #0 {
                    n231 = local write "Error Message"("MP can not be started.\nReason:*PL-VBV can be open. \n   *CH-VBV can be open." ("Error Message")) -> ()
                  }
                  frame #1 {
                    n232 = stacked-sequence {
                      frame #0 {
                        n233 = local write "Ch3_Pl_atm_do"(T/1 ("Ch1_Mp_do")) -> ()
                      }
                      frame #1 {
                        n234 = Wait (ms)(milliseconds to wait=i32? 1000) -> ()  [unwired: 1 out]
                      }
                      frame #2 {
                        n235 = local write "Ch3_Ch_atm_do"(T/1 ("Ch1_Mp_do")) -> ()
                      }
                      frame #3 {
                        n236 = Wait (ms)(milliseconds to wait=i32? 1000) -> ()  [unwired: 1 out]
                      }
                      frame #4 {
                        n237 = local write "Ch3_Mp_do"(T/1 ("Ch1_Mp_do")) -> ()
                      }
                    }
                  }
                }
              }
            }
            n238 = case shown="True" w1771 {
              frame #0 {
              }
              frame #1 {
                n239 = local read "Ch3_Mp_stop_safety"() -> (w1791)
                n240 = case shown="True" w1791 {
                  frame #0 {
                    n241 = local write "Error Message"("MP can not be stopped.\nReason :*TP-BV can be open." ("Error Message")) -> ()
                  }
                  frame #1 {
                    n242 = stacked-sequence {
                      frame #0 {
                        n243 = local write "Ch3_Mp_do"(i16? 0 ("Ch1_Mp_do")) -> ()
                      }
                      frame #1 {
                        n244 = Wait (ms)(milliseconds to wait=i32? 500) -> ()  [unwired: 1 out]
                      }
                      frame #2 {
                        n245 = local write "Ch3_Pl_atm_do"(i16? 0 ("Ch1_Mp_do")) -> ()
                      }
                      frame #3 {
                        n246 = Wait (ms)(milliseconds to wait=i32? 500) -> ()  [unwired: 1 out]
                      }
                      frame #4 {
                        n247 = local write "Ch3_Pl_vbv_do"(T/1 ("Ch1_Pl_vbv_do")) -> ()
                      }
                    }
                  }
                }
              }
            }
            n248 = Or(x="Ch4_Mp_stop_gui", y="Ch4_Mp_stop") -> (x .or. y?=w1754)
            n249 = Or(x="Ch4_Mp_start_gui", y="Ch4_Mp_start") -> (x .or. y?=w1757)
            n250 = case shown="True" w1757 {
              frame #0 {
              }
              frame #1 {
                n251 = local read "Ch4_Mp_start_safety"() -> (w1784)
                n252 = case shown="True" w1784 {
                  frame #0 {
                    n253 = local write "Error Message"("MP can not be started.\nReason:*PL-VBV can be open. \n   *CH-VBV can be open." ("Error Message")) -> ()
                  }
                  frame #1 {
                    n254 = stacked-sequence {
                      frame #0 {
                        n255 = local write "Ch4_Pl_atm_do"(T/1 ("Ch1_Mp_do")) -> ()
                      }
                      frame #1 {
                        n256 = Wait (ms)(milliseconds to wait=i32? 1000) -> ()  [unwired: 1 out]
                      }
                      frame #2 {
                        n257 = local write "Ch4_Ch_atm_do"(T/1 ("Ch1_Mp_do")) -> ()
                      }
                      frame #3 {
                        n258 = Wait (ms)(milliseconds to wait=i32? 1000) -> ()  [unwired: 1 out]
                      }
                      frame #4 {
                        n259 = local write "Ch4_Mp_do"(T/1 ("Ch1_Mp_do")) -> ()
                      }
                    }
                  }
                }
              }
            }
            n260 = case shown="True" w1754 {
              frame #0 {
              }
              frame #1 {
                n261 = local read "Ch4_Mp_stop_safety"() -> (w1777)
                n262 = case shown="True" w1777 {
                  frame #0 {
                    n263 = local write "Error Message"("MP can not be stopped.\nReason :*TP-BV can be open." ("Error Message")) -> ()
                  }
                  frame #1 {
                    n264 = stacked-sequence {
                      frame #0 {
                        n265 = local write "Ch4_Mp_do"(i16? 0 ("Ch1_Mp_do")) -> ()
                      }
                      frame #1 {
                        n266 = Wait (ms)(milliseconds to wait=i32? 500) -> ()  [unwired: 1 out]
                      }
                      frame #2 {
                        n267 = local write "Ch4_Pl_atm_do"(i16? 0 ("Ch1_Mp_do")) -> ()
                      }
                      frame #3 {
                        n268 = Wait (ms)(milliseconds to wait=i32? 500) -> ()  [unwired: 1 out]
                      }
                      frame #4 {
                        n269 = local write "Ch4_Pl_vbv_do"(T/1 ("Ch1_Pl_vbv_do")) -> ()
                      }
                    }
                  }
                }
              }
            }
          }
        }
        n270 = stacked-sequence {
          frame #0 {
            # "BUZZER DEACTIVE"
            n271 = case shown="True" "Buzzer_deactive" {
              frame #0 {
              }
              frame #1 {
                n272 = local write "Cnt_Do_Buzzer"(i16? 0 ("Cnt_Do_Buzzer")) -> ()
              }
            }
          }
        }
        n273 = stacked-sequence {
          frame #0 {
            n274 = stacked-sequence {
              frame #0 {
                n275 = case shown="True" "Ch1_Pet_cool_down" {
                  frame #0 {
                  }
                  frame #1 {
                    n276 = stacked-sequence {
                      frame #0 {
                        n277 = local write "Ch1_Pet_cool_up_do"(i16? 0 ("Ch1_Trns_gv_open_do")) -> ()
                      }
                      frame #1 {
                        n278 = local write "Ch1_Pet_cool_down_do"(T/1 ("Ch1_Trns_gv_open_do")) -> ()
                      }
                    }
                  }
                }
                n279 = case shown="True" "Ch1_Pet_cool_up" {
                  frame #0 {
                  }
                  frame #1 {
                    n280 = stacked-sequence {
                      frame #0 {
                        n281 = local write "Ch1_Pet_cool_down_do"(i16? 0 ("Ch1_Trns_gv_open_do")) -> ()
                      }
                      frame #1 {
                        n282 = local write "Ch1_Pet_cool_up_do"(T/1 ("Ch1_Trns_gv_open_do")) -> ()
                      }
                    }
                  }
                }
              }
            }
            n283 = case shown="True" "Ch1_Cst_fix_down" {
              frame #0 {
              }
              frame #1 {
                n284 = stacked-sequence {
                  frame #0 {
                    n285 = local write "Ch1_Cst_fix_do"(T/1 ("Ch1_Trns_gv_open_do")) -> ()